vi "ScanDelay_FTIR_BBnorm_Aligning_NewportFlipper.vi"() -> ()   [LabVIEW 2022 SP3]
uses:
  Control_scanDelayWorkflow.ctl
  Control_GetSpectrum_BBnorm.ctl
panel:
  in  "Power threshold":dbl(slide)=97.70099572992264 scale=10.0..1000.0
  in  "Update alignment":bool
  in  "Bright beam: alignment delay":i32=-12
  in  "Norm phase offset":dbl
  in  "Bright beam: physical channels (inputV, ScanDelay X)":tag="Dev1/ai2,Dev1/ai3"
  in  "Sample: physical channels (inputV, ScanDelay X)":tag="Dev1/ai6,Dev1/ai3"
  in  "Sample: alignment delay":i32=-1
  in  "Path to save\nnormalized spectrum":path=path "C:/Users/mnopl/Dropbox/Data/Park-SNOM/2022.08.21 - InSb nanowire/nanoFTIR/InSB nanowire norm gold, 2x integration.txt"
  in  "Save normalized\nspectrum":bool
  in  "Optimize\ninterferogram\nalignment":bool
  in  "Acquire only\nBB 100% curve with\nspoofed flip":bool
  in  "Toggle BB\nmirror\nUp / Down":bool
  in  "Realign phase":bool=TRUE
  in  "Recalibrate BB\nfrequency":bool
  in  "Pause\nacquisition":bool
  in  "Replicate\nfrom #":i8=4 min=0
  in  "Envelope width":dbl(slide)=1.878787878787879 scale=0.25..4.0
  out "Accumulated sample BB spectrum":dbl[][](array[numeric])
  out "Accumulated sample spectrum":dbl[][](array[numeric])
  in  "BB-reference spectrum":bool
  in  "Acquire only\nBB 100% curve":bool
  in  "Toggle pause (ms)":dbl=3000.0
  out "BB-referenced spectrum (phase)":T1(graph)={"Output spectrum"=[1913.547225668975, 1916.0355835697148, 1918.5239414704547, 1921.0122993711946, 1923.5006572719346, 1925.9890151726745, 1928.4773730734144, 1930.9657309741542, 1933.454088874894, 1935.942446775634, 1938.4308046763738, 1940.9191625771139, 1943.4075204778537, 1945.8958783785936, 1948.3842362793334, 1950.8725941800733, 1953.3609520808131, 1955.849309981553, 1958.337667882293, 1960.826025783033, 1963.3143836837728, 1965.8027415845127, 1968.2910994852525, 1970.7794573859924, 1973.2678152867322, 1975.7561731874723, 1978.2445310882122, 1980.732888988952, 1983.2212468896919, 1985.7096047904317, 1988.1979626911716, 1990.6863205919115, 1993.1746784926515, 1995.6630363933914, 1998.1513942941313, 2000.639752194871, 2003.128110095611, 2005.6164679963508, 2008.1048258970907, 2010.5931837978308, 2013.0815416985706, 2015.5698995993105, 2018.0582575000503, 2020.5466154007902, 2023.03497330153], "Output spectrum"=[-1.050141865778187, -1.0863175683631994, -0.688619248474197, -0.4185634136777594, -0.5646159369126735, -0.6022045865419159, -0.5994215462758917, -0.6066834140301581, -0.3137882972597481, -0.23139650643690857, -0.28989744609145873, -0.22766278995203496, -0.3072708379838787, -0.28807864115577786, -0.20144463008335833, -0.23846578437127167, -0.03358903801841962, -0.1680125942189079, -0.1754095156419453, -0.018688939519051935, -0.017175298030565504, -0.15591934166263854, -0.1833572707497524, -0.14414513056880193, -0.10541629799871545, -0.11890326964959286, -0.0942358420892333, -0.1092209107110307, -0.10121414288988718, -0.02851281346289625, -0.06429589239320421, -0.18827603842390775, -0.2841226664638725, -0.3030969989337109, -0.3233848660412946, -0.301291148807195, -0.1961849659955988, -0.2371140150369797, -0.3370162547967083, -0.49085440487078813, -0.5434984989709051, -0.4297745571172982, -0.46466561616671237, -0.5739202225203712, -0.9312624047314557]}
  out "BB-referenced spectrum (amplitude)":T2(graph)={"Sample Spectra"=[1913.547225668975, 1916.0355835697148, 1918.5239414704547, 1921.0122993711946, 1923.5006572719346, 1925.9890151726745, 1928.4773730734144, 1930.9657309741542, 1933.454088874894, 1935.942446775634, 1938.4308046763738, 1940.9191625771139, 1943.4075204778537, 1945.8958783785936, 1948.3842362793334, 1950.8725941800733, 1953.3609520808131, 1955.849309981553, 1958.337667882293, 1960.826025783033, 1963.3143836837728, 1965.8027415845127, 1968.2910994852525, 1970.7794573859924, 1973.2678152867322, 1975.7561731874723, 1978.2445310882122, 1980.732888988952, 1983.2212468896919, 1985.7096047904317, 1988.1979626911716, 1990.6863205919115, 1993.1746784926515, 1995.6630363933914, 1998.1513942941313, 2000.639752194871, 2003.128110095611, 2005.6164679963508, 2008.1048258970907, 2010.5931837978308, 2013.0815416985706, 2015.5698995993105, 2018.0582575000503, 2020.5466154007902, 2023.03497330153], "Sample Spectra"=[0.21431528991656407, 0.2217790309360323, 0.31059051804165827, 0.2559580093366482, 0.19394427644619502, 0.1870420437562703, 0.17940883999180368, 0.19737590618319079, 0.18493265337843712, 0.17072287627421948, 0.1885297071992416, 0.2166851592615681, 0.2045139777663893, 0.21994789452771624, 0.19933120098365714, 0.20847152851762896, 0.21733342018742194, 0.18201662025093124, 0.20345472411520035, 0.21816141432388855, 0.20539415711710124, 0.20171935426648782, 0.21982181204405915, 0.2210962336039931, 0.22055930529544074, 0.21195615084865987, 0.2203380461459153, 0.21465424994113436, 0.22568562951880414, 0.23567243763643142, 0.22689650039887704, 0.22001105660380255, 0.22812845633815412, 0.23960259569466802, 0.24398578523827416, 0.2672533752620745, 0.2689613845452476, 0.24882358351023065, 0.24547865050517487, 0.266249741497733, 0.3436542239006744, 0.369785092951132, 0.33663993490895827, 0.3315616535631962, 0.2820292556481605]}
  out "Reference BB spectra":dbl[][](array[numeric])
  out "Reference spectra":dbl[][](array[numeric])
  out "Latest replication cmd":string="@rep load 32"
  in  "Replicate\nalpha on\naccumulation":bool=TRUE
  out "# Accumulated":i32=1
  in  "Accumulate to #":i32=35
  in  "Cancel\nacquisition":bool
  out "Toggle position":i32=1
  out "Spectrum stored":bool
  out "Reference stored":bool
  out "Normalized spectrum (phase)":T1(graph)
  out "Normalized spectrum (amplitude)":T1(graph)
  in  "Store as reference":bool
  out "Python alpha rep path":path=path "C:/Users/mnopl/Desktop/software/mnOPSuite/PRISM/python/alpha.py"
  out "Activity status":string="Awaiting command"
  out "Acquisition status":string="Ready to acquire spectrum"
  in  "Path to save spectrum":path=path "C:/Users/mnopl/Dropbox/Data/Park-SNOM/2022.08.21 - InSb nanowire/nanoFTIR/InSb nanowire - 2x integration.txt"
  in  "Load reference":bool
  in  "Path to load reference":path=path "C:/Users/mnopl/Dropbox/Data/Park-SNOM/2022.08.20 - nanoFTIR on 100nm SiO2 - new beamsplitter/Si bulk reference, 700-1500 cm-1.txt"
  in  "Path to load spectrum":path=path "C:/Users/mnopl/Dropbox/Data/Park-SNOM/2022.08.21 - InSb nanowire/nanoFTIR/InSb nanowire 2.txt"
  in  "Apply spectral\nenvelope":bool=TRUE
  out "Binned interferogram":cluster{"X":dbl, "Y":dbl}[](graph)
  out "Sample BB Spectra":dbl[][](array[numeric])
  out "Sample Spectra":dbl[][](array[numeric])
  out "Python error: spectrum acquisition":errorcluster
  out "Python scandelay path":path=path "C:/Users/mnopl/Desktop/software/mnOPSuite/PRISM/python/scandelay_FTIR.py"
  in  "Time per\nacquisition (s)":dbl=0.18
  in  "Sampling rate":dbl=250000.0
  in  "Delay calibratior\nfactor (ps/V)":dbl=-2.495 format="%_6g"
  in  "Cycles per\ninterferogram":i32=50
  out "Accumulated spectrum (amplitude)":T3(graph)
  out "Acquisition cycle":dbl[][](graph)
  out "% averaged":dbl=100.0
  in  "Halt program":bool
  out "Python error: activity loop":errorcluster
  in  "Load spectrum":bool
  in  "Save spectrum":bool
  in  "Normalize spectrum":bool
  in  "Acquire spectrum":bool
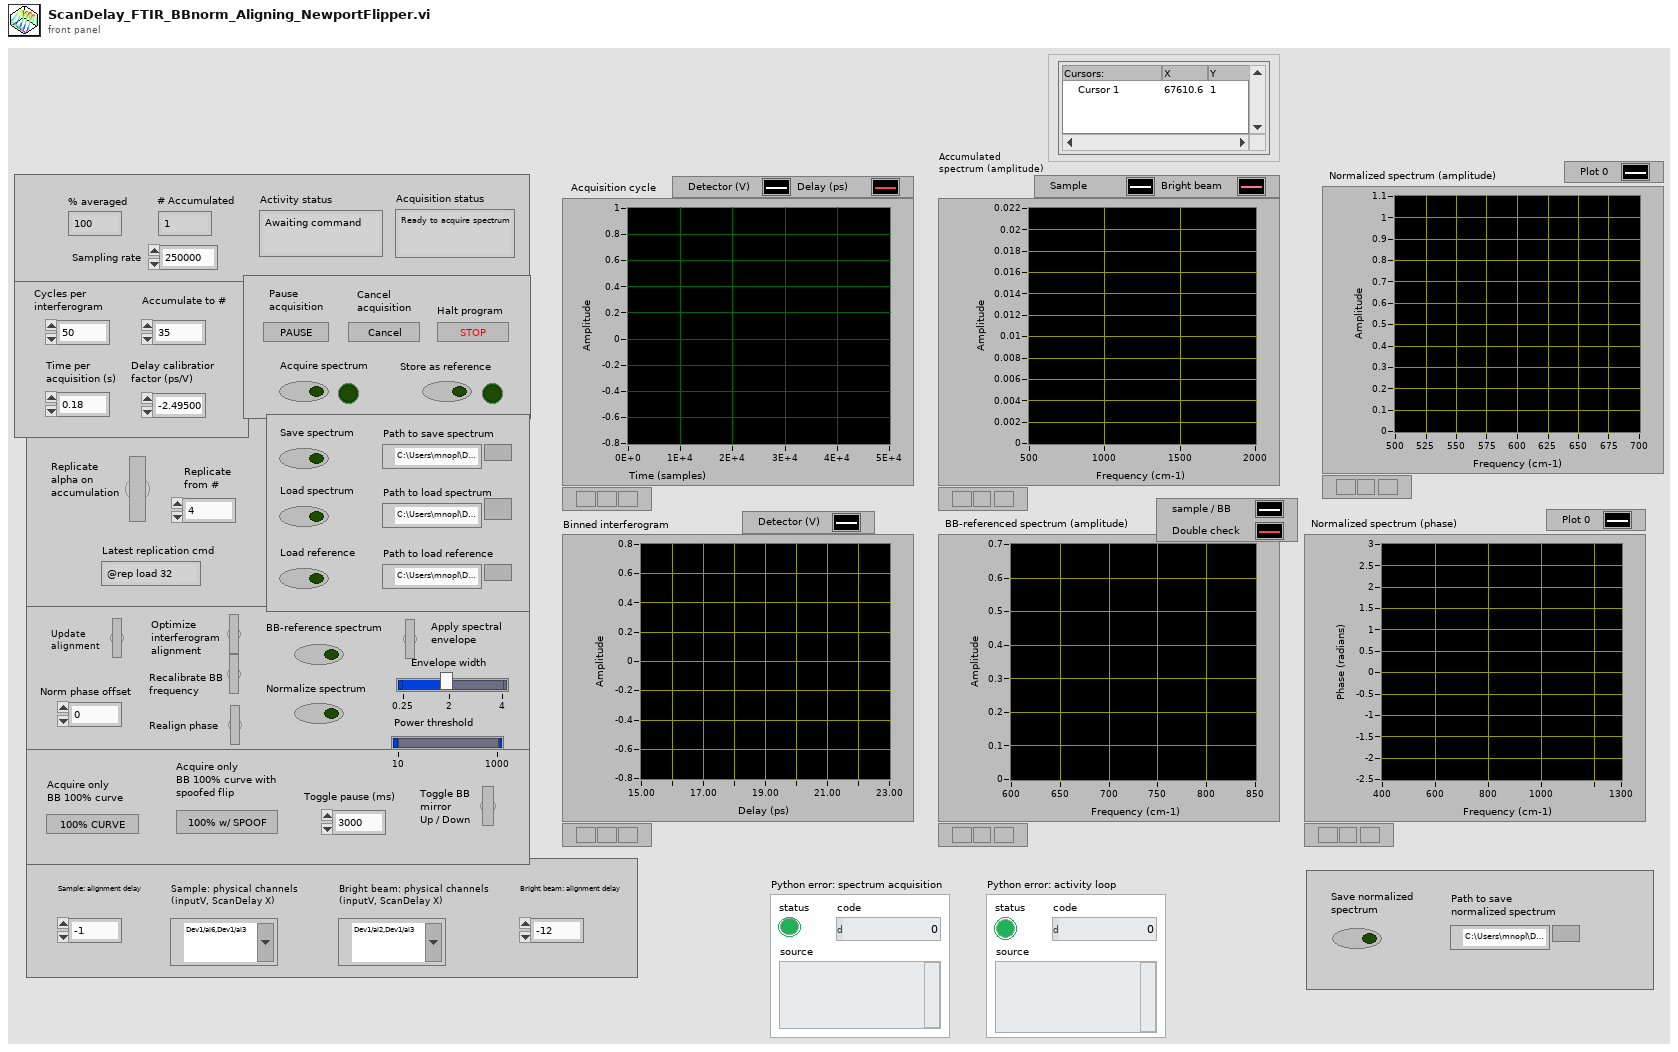
[diagram p1: front panel]
types:
  T1 = cluster{"Output spectrum":dbl[], "Output spectrum":dbl[]}
  T2 = cluster{"Sample Spectra":dbl[], "Sample Spectra":dbl[]}
  T3 = cluster{"Output spectrum":dbl[], "Output spectrum":dbl[]}[]
  T4 = typedef "Control_scanDelayWorkflow.ctl" = enum16{"Initialize", "Sit Idle", "Load replicator table", "Flip BB", "Load Spectrum", "Store reference", "Save Spectrum", "Load reference", "Check Reference", "Check Spectrum", "BB reference spectrum", "Normalize Spectrum", "Save normalized spectrum", "Done"}
  T5 = typedef "imagedata.ctl" = cluster{"image type":i32, "image depth":i32, "image":u8[], "mask":u8[], "colors":u32[], "Rectangle":cluster{"left":i16, "top":i16, "right":i16, "bottom":i16}}
  T6 = typedef "Control_GetSpectrum_BBnorm.ctl" = enum16{"Initialize", "Replicate alpha", "Flip in BB", "Get Spectrum", "Accumulate BB spectrum", "Flip out BB", "Accumulate sample spectrum", "Assess accumulation", "Finalize", "Done"}
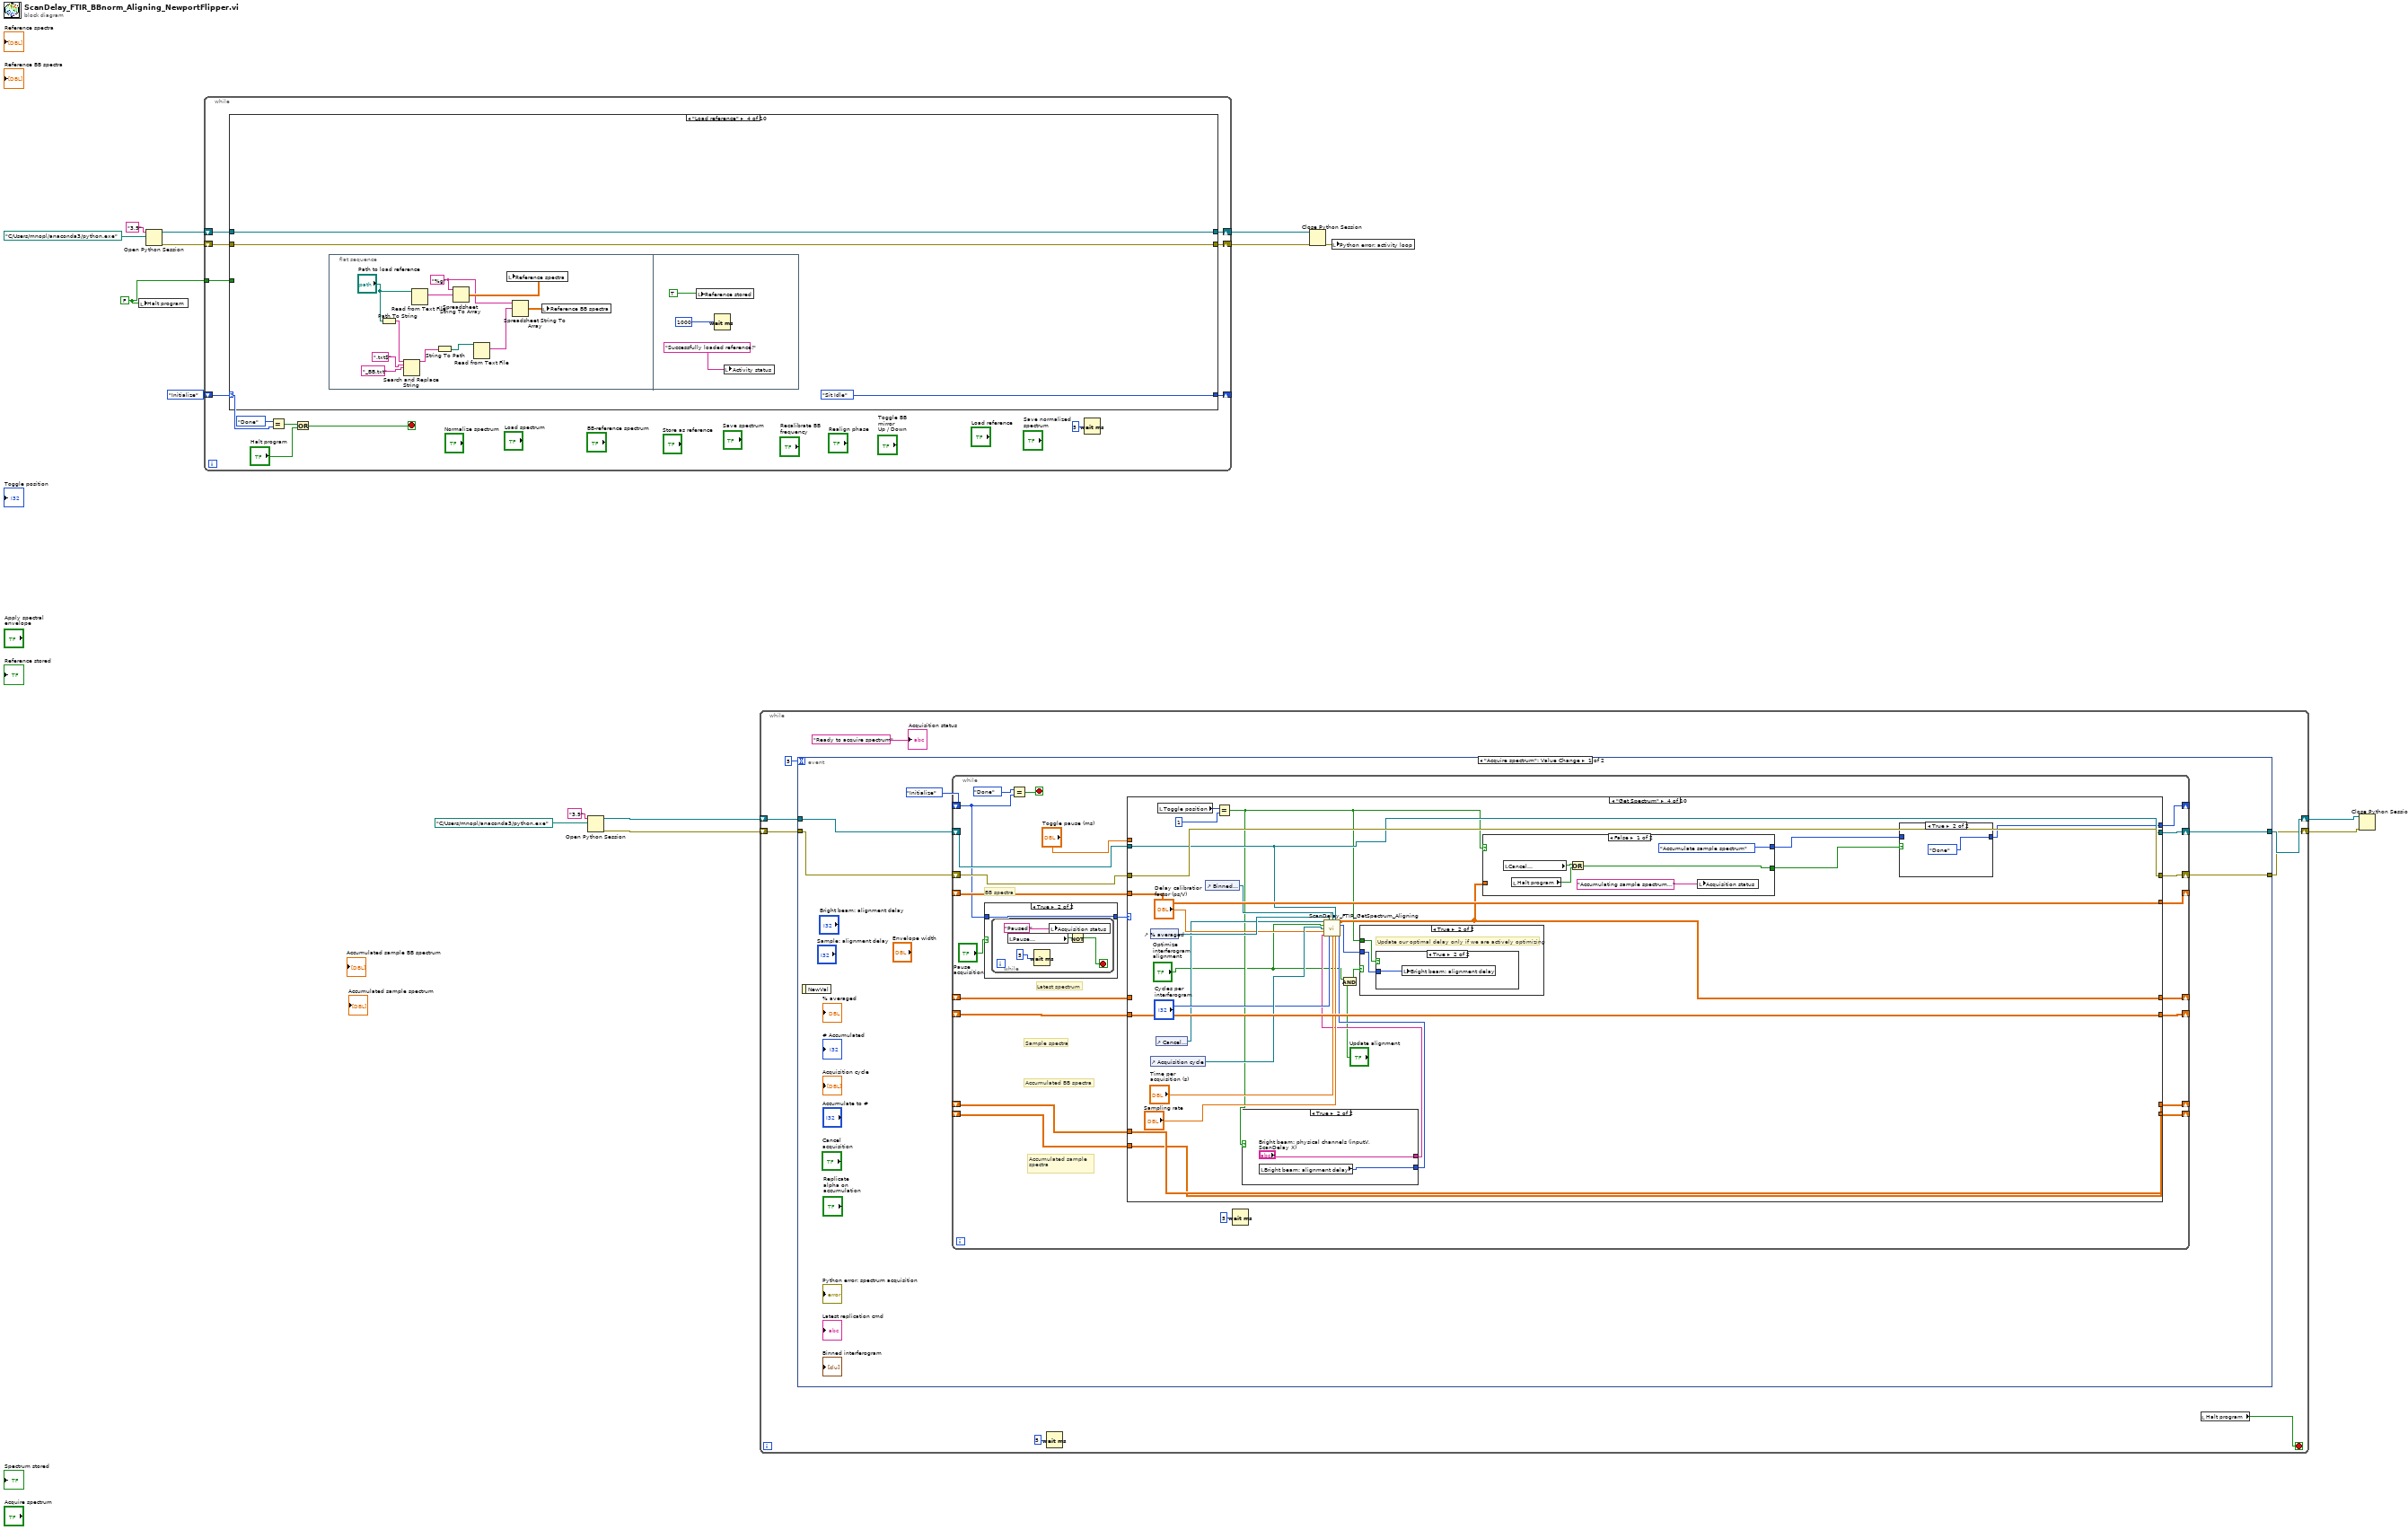
[diagram p0: block diagram]
diagram:
  w1 = FALSE
  n1 = local write "Halt program"(w1) -> ()
  n2 = Open Python Session(python version="3.9", python path=path "C:/Users/mnopl/anaconda3/python.exe") -> (session out=w11:refnum<k35>, error out=w10:errorcluster)  [unwired: 1 in]
  n3 = while {
    shift-right: [w20] -> _
    shift-left: Control_scanDelayWorkflow."Initialize" -> [w17]
    shift-right: [w26] -> w12
    shift-left: w10 -> [w18]
    shift-right: [w21] -> w13
    shift-left: w11 -> [w19]
    tunnel: w1 -> [w16]
    stop <- w24 stop-if-true
    n4 = case shown="\"Load reference\"" w17 {
      tunnel: [w31 w70 w80 w99 w120 w169 w188 w200 w243 w250] -> w26
      tunnel: w19 -> [w32 w69 w79 w100 w123 w170 w189 w198 w244 w251]
      tunnel: w18 -> [w31 w70 w80 w99 w122 w169 w188 w197 w243 w250]
      tunnel: [w32 w69 w79 w100 w121 w170 w189 w199 w244 w251] -> w21
      tunnel: [w30 Control_scanDelayWorkflow."Sit Idle" Control_scanDelayWorkflow."Sit Idle" Control_scanDelayWorkflow."Sit Idle" Control_scanDelayWorkflow."Sit Idle" Control_scanDelayWorkflow."Sit Idle" Control_scanDelayWorkflow."Sit Idle" Control_scanDelayWorkflow."Sit Idle" Control_scanDelayWorkflow."Sit Idle" Control_scanDelayWorkflow."Sit Idle"] -> w20
      tunnel: w16 -> [_ _ _ _ _ _ w185 _ _ _]
      frame "Sit Idle", Default {
        n5 = event shown="[4] \"Save normalized spectrum\": Value Change" {
          selector: _ -> [_ _ _ _ _ _ _ _ _]
          dyn-events: _ -> [_ _ _ _ _ _ _ _ _]
          timeout: 5 -> [_ _ _ _ _ _ _ _ w62]
          tunnel: [w33 w37 w44 Control_scanDelayWorkflow."Flip BB" w46 w50 w54 w58 Control_scanDelayWorkflow."Sit Idle"] -> w30
          event "Normalize spectrum": Value Change {
            n6 = event-data() -> ("NewVal"=w34:bool)  [unwired: 1 in]
            n7 = Select(t=Control_scanDelayWorkflow."Normalize Spectrum", s=w34, f=Control_scanDelayWorkflow."Sit Idle") -> (s? t:f=w33:T4)
          }
          event "Store as reference": Value Change {
            n8 = event-data() -> ("NewVal"=w40:bool)  [unwired: 1 in]
            n9 = Select(t=Control_scanDelayWorkflow."Store reference", s=w40, f=Control_scanDelayWorkflow."Sit Idle") -> (s? t:f=w37:T4)
          }
          event "BB-reference spectrum": Value Change {
            n10 = event-data() -> ("NewVal"=w42:bool)  [unwired: 1 in]
            n11 = Select(t=Control_scanDelayWorkflow."BB reference spectrum", s=w42, f=Control_scanDelayWorkflow."Sit Idle") -> (s? t:f=w44:T4)
          }
          event "Toggle BB\nmirror\nUp / Down": Value Change {
            n12 = event-data() -> ()  [unwired: 1 in, 1 out]
          }
          event "Save normalized\nspectrum": Value Change {
            n13 = event-data() -> ("NewVal"=w47:bool)  [unwired: 1 in]
            n14 = Select(t=Control_scanDelayWorkflow."Save normalized spectrum", s=w47, f=Control_scanDelayWorkflow."Sit Idle") -> (s? t:f=w46:T4)
          }
          event "Save spectrum": Value Change {
            n15 = event-data() -> ("NewVal"=w51:bool)  [unwired: 1 in]
            n16 = Select(t=Control_scanDelayWorkflow."Save Spectrum", s=w51, f=Control_scanDelayWorkflow."Sit Idle") -> (s? t:f=w50:T4)
          }
          event "Load reference": Value Change {
            n17 = event-data() -> ("NewVal"=w57:bool)  [unwired: 1 in]
            n18 = Select(t=Control_scanDelayWorkflow."Load reference", s=w57, f=Control_scanDelayWorkflow."Sit Idle") -> (s? t:f=w54:T4)
          }
          event "Load spectrum": Value Change {
            n19 = event-data() -> ("NewVal"=w59:bool)  [unwired: 1 in]
            n20 = Select(t=Control_scanDelayWorkflow."Load Spectrum", s=w59, f=Control_scanDelayWorkflow."Sit Idle") -> (s? t:f=w58:T4)
          }
          event Timeout {
            n21 = event-data() -> ()  [unwired: 1 in, 2 out]
            n22 = Wait (ms)(milliseconds to wait=w62) -> ()  [unwired: 1 out]
          }
        }
        "Activity status" <- "Awaiting command"
      }
      frame "Store reference" {
        # "Is spectrum a full array?"
        n23 = local read "Sample Spectra"() -> (w65:dbl[][])
        n24 = local read "Sample BB Spectra"() -> (w64:dbl[][])
        n25 = Empty Array?(array=w65) -> (empty?=w67:bool)
        n26 = Not(x=w67) -> (.not. x?=w66:bool)
        n27 = case shown="True" w66 {
          tunnel: w65 -> [_ w73]
          tunnel: w64 -> [_ w74]
          frame False {
            n28 = Wait (ms)(milliseconds to wait=1000) -> ()  [unwired: 1 out]
            n29 = local write "Activity status"("Error: Spectrum is empty!") -> ()
          }
          frame True {
            n30 = local write "Reference BB spectra"(w74) -> ()
            n31 = local write "Reference spectra"(w73) -> ()
            n32 = local write "Reference stored"(TRUE) -> ()
            n33 = Wait (ms)(milliseconds to wait=1000) -> ()  [unwired: 1 out]
            n34 = local write "Activity status"("Storing reference!") -> ()
          }
        }
      }
      frame "Save Spectrum" {
        n35 = flat-sequence {
          frame #0 {
            w86 = "%g"
            n36 = local read "Sample Spectra"() -> (w88:dbl[][])
            n37 = Path To String(path="Path to save spectrum") -> (string=w90:string)
            n38 = local read "Sample BB Spectra"() -> (w81:dbl[][])
            n39 = Search and Replace String(input string=w90, search string="(.txt)*$", replace string=".txt") -> (result string=w94:string)  [unwired: 5 in, 3 out]
            n40 = Search and Replace String(input string=w94, search string=".txt$", replace string="_BB.txt") -> (result string=w93:string)  [unwired: 5 in, 3 out]
            n41 = String To Path(string=w94) -> (path=w91:path)
            n42 = Array To Spreadsheet String(array=w88, 3:w86) -> (spreadsheet string=w87:string)  [unwired: 1 in]
            n43 = Array To Spreadsheet String(array=w81, 3:w86) -> (spreadsheet string=w95:string)  [unwired: 1 in]
            n44 = String To Path(string=w93) -> (path=w92:path)
            n45 = Write to Text File(file (use dialog)=w91, text=w87) -> ()  [unwired: 2 in, 3 out]
            n46 = Write to Text File(file (use dialog)=w92, text=w95) -> ()  [unwired: 2 in, 3 out]
          }
          frame #1 {
            n47 = local write "Activity status"("Successfully saved spectrum!") -> ()
            n48 = Wait (ms)(milliseconds to wait=1000) -> ()  [unwired: 1 out]
          }
        }
      }
      frame "Load reference" {
        n49 = flat-sequence {
          frame #0 {
            w105 = "%g"
            n50 = Path To String(path="Path to load reference") -> (string=w101:string)
            n51 = Search and Replace String(input string=w101, search string=".txt$", replace string="_BB.txt") -> (result string=w103:string)  [unwired: 5 in, 3 out]
            n52 = Read from Text File(file (use dialog)="Path to load reference") -> (text=w106:string)  [unwired: 3 in, 3 out]
            n53 = String To Path(string=w103) -> (path=w110:path)
            n54 = Spreadsheet String To Array(format string=w105, spreadsheet string=w106) -> (array=w107:dbl[][])  [unwired: 2 in]
            n55 = Read from Text File(file (use dialog)=w110) -> (text=w109:string)  [unwired: 3 in, 3 out]
            n56 = local write "Reference spectra"(w107) -> ()
            n57 = Spreadsheet String To Array(format string=w105, spreadsheet string=w109) -> (array=w111:dbl[][])  [unwired: 2 in]
            n58 = local write "Reference BB spectra"(w111) -> ()
          }
          frame #1 {
            n59 = local write "Reference stored"(TRUE) -> ()
            n60 = Wait (ms)(milliseconds to wait=1000) -> ()  [unwired: 1 out]
            n61 = local write "Activity status"("Successfully loaded reference!") -> ()
          }
        }
      }
      frame "Normalize Spectrum" {
        n62 = local read "Reference stored"() -> (w117:bool)
        n63 = local read "Spectrum stored"() -> (w116:bool)
        n64 = And(x=w116, y=w117) -> (x .and. y?=w115:bool)
        n65 = flat-sequence {
          tunnel: w123 -> [w129]
          tunnel: w122 -> [w128]
          tunnel: [w127] -> w119
          tunnel: [w126] -> w118
          tunnel: w115 -> [w125]
          tunnel: [w166] -> w120
          tunnel: [w167] -> w121
          tunnel: w119 -> [w167]
          tunnel: w118 -> [w166]
          frame #0 {
            n66 = case shown="True" w125 {
              tunnel: w129 -> [w131 w163]
              tunnel: w128 -> [w130 w162]
              tunnel: [w131 w161] -> w127
              tunnel: [w130 w144] -> w126
              frame False {
                n67 = Wait (ms)(milliseconds to wait=1000) -> ()  [unwired: 1 out]
                n68 = local write "Activity status"("Error: Spectrum or reference is empty!") -> ()
              }
              frame True {
                n69 = Wait (ms)(milliseconds to wait=1000) -> ()  [unwired: 1 out]
                n70 = local read "Python scandelay path"() -> (w160:path)
                n71 = local read "Sample Spectra"() -> (w145:dbl[][])
                n72 = local read "Sample BB Spectra"() -> (w146:dbl[][])
                n73 = local read "Reference spectra"() -> (w143:dbl[][])
                n74 = local read "Reference BB spectra"() -> (w142:dbl[][])
                n75 = local read "Apply spectral\nenvelope"() -> (w141:bool)
                n76 = local read "Envelope width"() -> (w140:dbl)
                n77 = local read "Recalibrate BB\nfrequency"() -> (w139:bool)
                n78 = local read "Realign phase"() -> (w138:bool)
                n79 = local write "Activity status"("Normalizing spectrum!") -> ()
                n80 = Divide(x=1, y="Power threshold") -> (x/y=w134:dbl)
                n81 = node(w163, w160, "normalized_spectrum", w162, w145, w145, w146, w143, w142, w141, w140, w139, w138, "Norm phase offset", w134) -> (w161:refnum<k35>, w144:errorcluster, w148:dbl[][])  [unwired: 10 in, 2 out]
                "Python error: activity loop" <- w144
                n82 = Index Array(array=w148, index (row) #1=0, index (row) #2=1) -> (element #1=w156:dbl[], element #2=w155:dbl[])  [unwired: 2 in]
                n83 = Index Array(array=w148, index (row) #1=0, index (row) #2=2) -> (element #1=w152:dbl[], element #2=w151:dbl[])  [unwired: 2 in]
                n84 = Bundle("Sample Spectra"=w156, "Sample Spectra"=w155) -> (→"Normalized spectrum (amplitude)":T2)  [unwired: 1 in]
                n85 = Bundle("Sample Spectra"=w152, "Sample Spectra"=w151) -> (→"Normalized spectrum (phase)":T2)  [unwired: 1 in]
              }
            }
          }
          frame #1 {
            n86 = local write "Normalize spectrum"(FALSE) -> ()
          }
        }
      }
      frame "Load Spectrum" {
        n87 = flat-sequence {
          frame #0 {
            w178 = "%g"
            n88 = Path To String(path="Path to load spectrum") -> (string=w174:string)
            n89 = Search and Replace String(input string=w174, search string=".txt$", replace string="_BB.txt") -> (result string=w176:string)  [unwired: 5 in, 3 out]
            n90 = Read from Text File(file (use dialog)="Path to load spectrum") -> (text=w179:string)  [unwired: 3 in, 3 out]
            n91 = String To Path(string=w176) -> (path=w181:path)
            n92 = Spreadsheet String To Array(format string=w178, spreadsheet string=w179) -> (array=w172:dbl[][])  [unwired: 2 in]
            n93 = Read from Text File(file (use dialog)=w181) -> (text=w180:string)  [unwired: 3 in, 3 out]
            n94 = Spreadsheet String To Array(format string=w178, spreadsheet string=w180) -> (array=w171:dbl[][])  [unwired: 2 in]
            n95 = local write "Sample Spectra"(w172) -> ()
            n96 = local write "Sample BB Spectra"(w171) -> ()
          }
          frame #1 {
            n97 = local write "Spectrum stored"(TRUE) -> ()
            n98 = local write "Activity status"("Successfully loaded spectrum!") -> ()
            n99 = Wait (ms)(milliseconds to wait=1000) -> ()  [unwired: 1 out]
          }
        }
      }
      frame "Initialize" {
        n100 = local write "Reference stored"(w185) -> ()
        n101 = local write "Spectrum stored"(w185) -> ()
        n102 = local write "Acquire spectrum"(w185) -> ()
        "Python scandelay path" <- path "C:/Users/mnopl/Desktop/software/mnOPSuite/PRISM/python/scandelay_FTIR.py"
        "Python alpha rep path" <- path "C:/Users/mnopl/Desktop/software/mnOPSuite/PRISM/python/alpha.py"
      }
      frame "BB reference spectrum" {
        # "Is spectrum a full array?"
        n103 = local read "Sample Spectra"() -> (w191:dbl[][])
        n104 = Empty Array?(array=w191) -> (empty?=w193:bool)
        n105 = Not(x=w193) -> (.not. x?=w192:bool)
        n106 = flat-sequence {
          tunnel: w198 -> [w204]
          tunnel: w197 -> [w203]
          tunnel: w192 -> [w202]
          tunnel: [w206] -> w195
          tunnel: [w205] -> w194
          tunnel: w191 -> [w201]
          tunnel: [w240] -> w199
          tunnel: [w241] -> w200
          tunnel: w195 -> [w241]
          tunnel: w194 -> [w240]
          frame #0 {
            n107 = case shown="True" w202 {
              tunnel: [w207 w218] -> w206
              tunnel: [w208 w219] -> w205
              tunnel: w204 -> [w208 w228]
              tunnel: w203 -> [w207 w227]
              tunnel: w201 -> [_ w223]
              frame False {
                n108 = Wait (ms)(milliseconds to wait=1000) -> ()  [unwired: 1 out]
                n109 = local write "Activity status"("Error: Spectrum or reference is empty!") -> ()
              }
              frame True {
                n110 = local read "Python scandelay path"() -> (w222:path)
                n111 = local read "Sample BB Spectra"() -> (w226:dbl[][])
                n112 = local read "Apply spectral\nenvelope"() -> (w217:bool)
                n113 = local read "Envelope width"() -> (w216:dbl)
                n114 = local read "Recalibrate BB\nfrequency"() -> (w215:bool)
                n115 = local read "Realign phase"() -> (w214:bool)
                n116 = Wait (ms)(milliseconds to wait=1000) -> ()  [unwired: 1 out]
                n117 = local write "Activity status"("Referencing spectrum to bright beam...") -> ()
                n118 = local read "Power threshold"() -> (w212:dbl)
                n119 = Divide(x=1, y=w212) -> (x/y=w211:dbl)
                n120 = node(w228, w222, "BB_referenced_spectrum", w227, w223, w223, w226, w217, w216, w215, w214, w211) -> (w219:refnum<k35>, w218:errorcluster, w233:dbl[][])  [unwired: 7 in, 2 out]
                n121 = local write "Python error: activity loop"(w218) -> ()
                n122 = Index Array(array=w233, index (row) #1=0, index (row) #2=2) -> (element #1=w236:dbl[], element #2=w235:dbl[])  [unwired: 2 in]
                n123 = Index Array(array=w233, index (row) #1=0, index (row) #2=1) -> (element #1=w238:dbl[], element #2=w237:dbl[])  [unwired: 2 in]
                n124 = Bundle("Sample Spectra"=w236, "Sample Spectra"=w235) -> (→"BB-referenced spectrum (phase)":T2)  [unwired: 1 in]
                n125 = Bundle("Sample Spectra"=w238, "Sample Spectra"=w237) -> (→"BB-referenced spectrum (amplitude)":T2)  [unwired: 1 in]
              }
            }
          }
          frame #1 {
            n126 = local write "BB-reference spectrum"(FALSE) -> ()
          }
        }
      }
      frame "Flip BB" {
        n127 = local read "Toggle BB\nmirror\nUp / Down"() -> (w246:bool)
        n128 = local read "Toggle pause (ms)"() -> (w242:dbl)
        n129 = call "NewportFlipper.vi"("Settle time (ms)"=w242, "Up/Down"=w246) -> ()  [unwired: 10 in]
      }
      frame "Save normalized spectrum" {
        n130 = flat-sequence {
          tunnel: [w265] -> w252
          tunnel: [w253] -> w247
          tunnel: w252 -> [w279]
          tunnel: [w276] -> w248
          tunnel: w247 -> [w276]
          tunnel: w248 -> [w288]
          frame #0 {
            w270 = "%g"
            n131 = Path To String(path="Path to save\nnormalized spectrum") -> (string=w265:string)
            n132 = property on="Normalized spectrum (phase)" class="XYGraph (strict)"() -> ("Value"=w255:T1)  [unwired: 2 in, 2 out]
            n133 = property on="Normalized spectrum (amplitude)" class="XYGraph (strict)"() -> ("Value"=w263:T1)  [unwired: 2 in, 2 out]
            n134 = Unbundle(w263) -> ("Output spectrum"=w262:dbl[], "Output spectrum"=w261:dbl[])
            n135 = Unbundle(w255) -> ("Output spectrum"=w258:dbl[], "Output spectrum"=w257:dbl[])
            n136 = Build Array(w262, w261) -> (w260:dbl[][])
            n137 = Build Array(w258, w257) -> (w256:dbl[][])
            n138 = Search and Replace String(input string=w265, search string="(.txt)$", replace string="_normalized_phase.txt") -> (result string=w274:string)  [unwired: 5 in, 3 out]
            n139 = Search and Replace String(input string=w265, search string="(.txt)*$", replace string="_normalized_amplitude.txt") -> (result string=w253:string)  [unwired: 5 in, 3 out]
            n140 = Transpose 2D Array(2D array=w260) -> (transposed array=w259:dbl[][])
            n141 = Transpose 2D Array(2D array=w256) -> (transposed array=w254:dbl[][])
            n142 = Array To Spreadsheet String(array=w259, 3:w270) -> (spreadsheet string=w275:string)  [unwired: 1 in]
            n143 = Array To Spreadsheet String(array=w254, 3:w270) -> (spreadsheet string=w271:string)  [unwired: 1 in]
            n144 = String To Path(string=w274) -> (path=w273:path)
            n145 = String To Path(string=w253) -> (path=w272:path)
            n146 = Write to Text File(file (use dialog)=w273, text=w275) -> ()  [unwired: 2 in, 3 out]
            n147 = Write to Text File(file (use dialog)=w272, text=w271) -> ()  [unwired: 2 in, 3 out]
          }
          frame #1 {
            n148 = invoke on="Normalized spectrum (amplitude)" class="XYGraph (strict)" method="Get Image"() -> ("image data"=w278:T5)  [unwired: 6 in, 5 out]
            n149 = Search and Replace String(input string=w279, search string="(.txt)$", replace string="_normalized_amplitude.png") -> (result string=w285:string)  [unwired: 5 in, 3 out]
            n150 = String To Path(string=w285) -> (path=w284:path)
            n151 = call <vilib>:"Write PNG File.vi"("image data"=w278, "path to PNG file"=w284) -> ()  [unwired: 8 in, 2 out]
            n152 = invoke on="Normalized spectrum (phase)" class="XYGraph (strict)" method="Get Image"() -> ("image data"=w277:T5)  [unwired: 6 in, 5 out]
            n153 = Search and Replace String(input string=w279, search string="(.txt)$", replace string="_normalized_phase.png") -> (result string=w281:string)  [unwired: 5 in, 3 out]
            n154 = String To Path(string=w281) -> (path=w280:path)
            n155 = call <vilib>:"Write PNG File.vi"("image data"=w277, "path to PNG file"=w280) -> ()  [unwired: 8 in, 2 out]
          }
          frame #2 {
            n156 = local write "Save normalized\nspectrum"(FALSE) -> ()
            n157 = Concatenate Strings("Spectrum successfully saved to:" ("message"), "\r", w288) -> (w291:string)
            n158 = One Button Dialog(message=w291, button name ("OK")="OK") -> ()  [unwired: 1 out]
          }
        }
      }
    }
    n159 = Equal?(x=Control_scanDelayWorkflow."Done", y=w17) -> (x = y?=w22:bool)
    n160 = Or(x=w22, y="Halt program") -> (x .or. y?=w24:bool)
    n161 = Wait (ms)(milliseconds to wait=5) -> ()  [unwired: 1 out]
  }
  n162 = Open Python Session(python version="3.9", python path=path "C:/Users/mnopl/anaconda3/python.exe") -> (session out=w5:refnum<k35>, error out=w4:errorcluster)  [unwired: 1 in]
  n163 = while {
    shift-right: [w294] -> w2
    shift-left: w4 -> [w296]
    shift-right: [w295] -> w3
    shift-left: w5 -> [w297]
    stop <- w301 stop-if-true
    n164 = event shown="[0] \"Acquire spectrum\": Value Change" {
      selector: _ -> [_ _]
      dyn-events: _ -> [_ _]
      timeout: 5 -> [_ w562]
      tunnel: w297 -> [w305 w561]
      tunnel: w296 -> [w304 w560]
      tunnel: [w303 w561] -> w295
      tunnel: [w302 w560] -> w294
      event "Acquire spectrum": Value Change {
        n165 = event-data() -> ()  [unwired: 1 in, 1 out]
        n166 = while {
          shift-right: [w326] -> _
          shift-left: _ -> [w325]
          shift-right: [w327] -> _
          shift-left: _ -> [w324]
          shift-right: [w323] -> _
          shift-left: Control_GetSpectrum_BBnorm."Initialize" -> [w309]
          shift-right: [w320] -> w302
          shift-left: w304 -> [w321]
          shift-right: [w319] -> w303
          shift-left: w305 -> [w322]
          shift-right: [w318] -> _
          shift-left: _ -> [w316]
          shift-right: [w314] -> _
          shift-left: _ -> [w312]
          shift-right: [w313] -> _
          shift-left: _ -> [w311]
          stop <- w307 stop-if-true
          # "BB spectra"
          # "Accumulated BB spectra"
          # "Accumulated sample spectra"
          # "Sample spectra"
          # "Latest spectrum"
          n167 = case shown="True" "Pause\nacquisition" {
            tunnel: w309 -> [w329 w330]
            tunnel: [w329 w330] -> w308
            frame False {
            }
            frame True {
              n168 = while {
                stop <- w334 stop-if-true
                n169 = local read "Pause\nacquisition"() -> (w333:bool)
                n170 = Wait (ms)(milliseconds to wait=5) -> ()  [unwired: 1 out]
                n171 = local write "Acquisition status"("Paused!") -> ()
                n172 = Not(x=w333) -> (.not. x?=w334:bool)
              }
            }
          }
          n173 = Equal?(x=Control_GetSpectrum_BBnorm."Done", y=w309) -> (x = y?=w307:bool)
          n174 = case shown="\"Get Spectrum\"" w308 {
            tunnel: [w335 w363 w369 w404 w434 w471 w495 w517 w544 w555] -> w327
            tunnel: [w335 w364 w370 w403 w447 w472 w488 w518 w543 w557] -> w326
            tunnel: w325 -> [_ w364 w370 w403 w456 w472 w488 w518 w543 w557]